vi "Video Detection.vi"() -> ()   [LabVIEW 2020]
doc: "Filtr detected objects and return only cars. Returns also the coordiantes of the nearest one."
uses:
  <vilib>/vision/Deep Learning.llb/IMAQ DL Model Type.ctl
  <vilib>/userDefined/High Color/IMAQdx.ctl
  <vilib>/vision/Avi.llb/IMAQ AVI2 Refnum.ctl
  <vilib>/vision/Avi.llb/IMAQ AVI2 Codec Path.ctl
  <vilib>/vision/Deep Learning.llb/IMAQ DL Model Detect Objects Node Names.ctl
  <vilib>/vision/Deep Learning.llb/IMAQ DL Model Label.ctl
  <vilib>/vision/NI_Vision_Development_Module.lvlib
  <vilib>/vision/driver/NI_Vision_Acquisition_Software.lvlib
  <resource>/objmgr/imaqdx.rc
panel:
  out "fps detection":dbl
  out "Replay mode":bool
  in  "Turn on the replay mode":bool
  in  "?":T1(tab)
  in  "Camera Name":refnum<k21> caption="IMAQdx Session"
  out "fps cam":dbl
  out "height":u32
  out "width":u32
  in  "Start Frame Number":u32
  out "Frame Number":u32
  in  "Frame increment":i32=1
  in  "Video fps":u32=30
  in  "Video filename":string="test_moving2.avi"
  in  "Height":i32=1080
  in  "Width":i32=1920
  out "Distance":sgl(graph)
  out "Cars found":i32
  out "Car found":bool
  in  "Minimum Score Threshold":sgl=0.3 min=0 max=1 step=0.1 format="%.3g"
  out "Actual frame":T2(plugin-control)
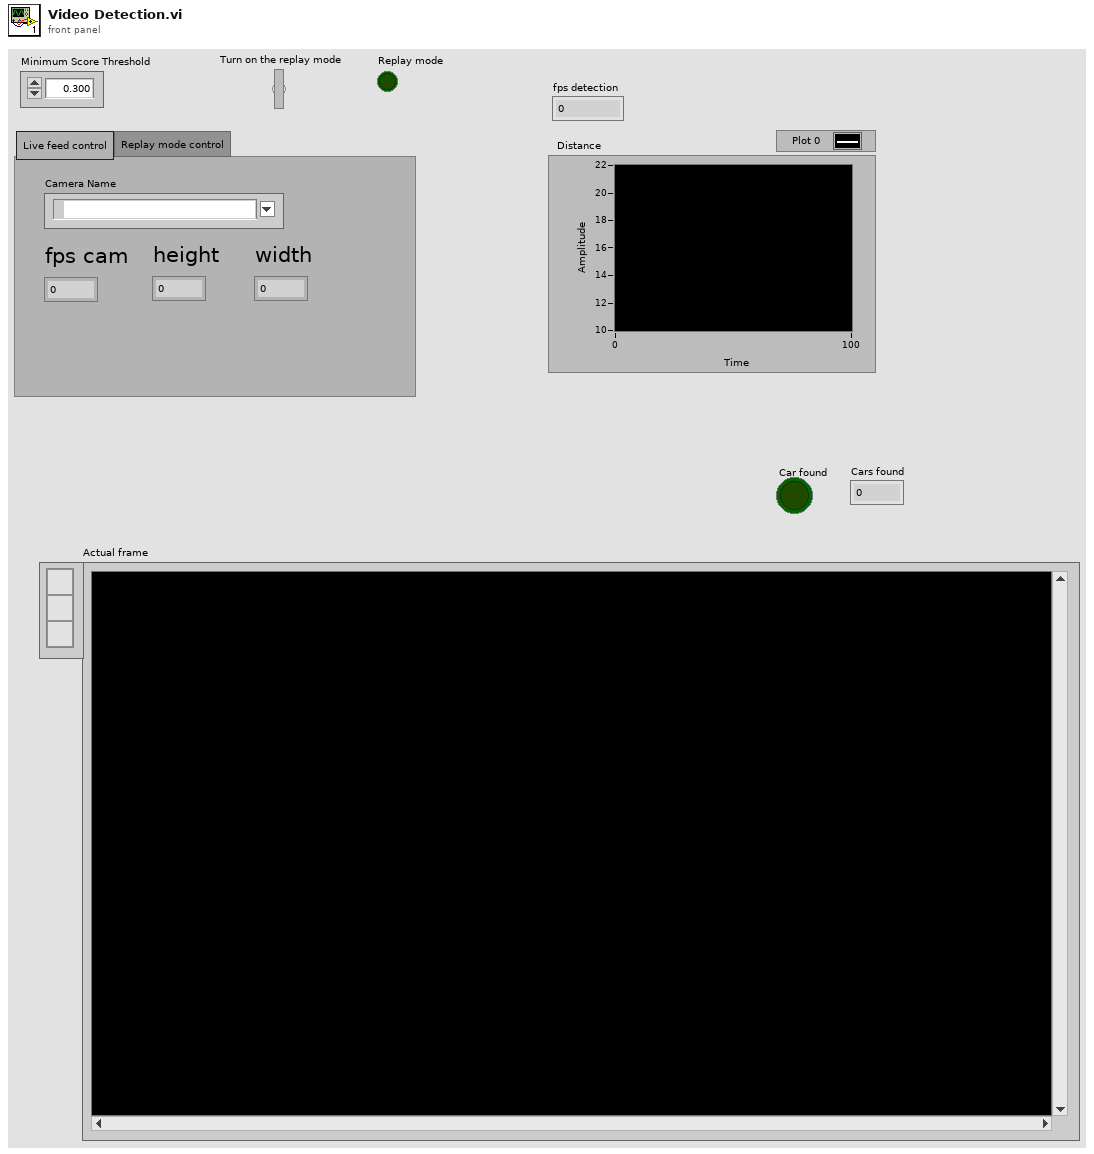
[diagram p1: front panel]
types:
  T1 = enum32{"Live feed control", "Replay mode control"}
  T2 = typedef "IMAQ Image.ctl" = refnum<image>
  T3 = typedef "IMAQdx.ctl" = refnum<k21>
  T4 = typedef "IMAQ AVI2 Refnum.ctl" = refnum<k20>
  T5 = typedef "IMAQ DL Model Type.ctl" = i32
  T6 = typedef "Image Type" = u32
  T7 = typedef "IMAQ AVI2 Codec Path.ctl" = u32
  T8 = typedef "IMAQ DL Model Refnum.ctl" = refnum<k20>
  T9 = typedef "IMAQ DL Model Label.ctl" = cluster{"ID":u32, "Label":string}
  T10 = typedef "IMAQ DL Model Detect Objects Node Names.ctl" = cluster{"Number of Objects":string, "Labels":string, "Scores":string, "Bounding Boxes":string}
  T11 = typedef "IMAQ DL Model Output Data.ctl" = cluster{"Node Name":string, "Data":sgl[], "Dimensions":u64[]}
  T12 = typedef "IMAQ DL Model Objects.ctl" = cluster{"Label":string, "Score":sgl, "Bounding Box":cluster{"x":sgl, "y":sgl}[]}
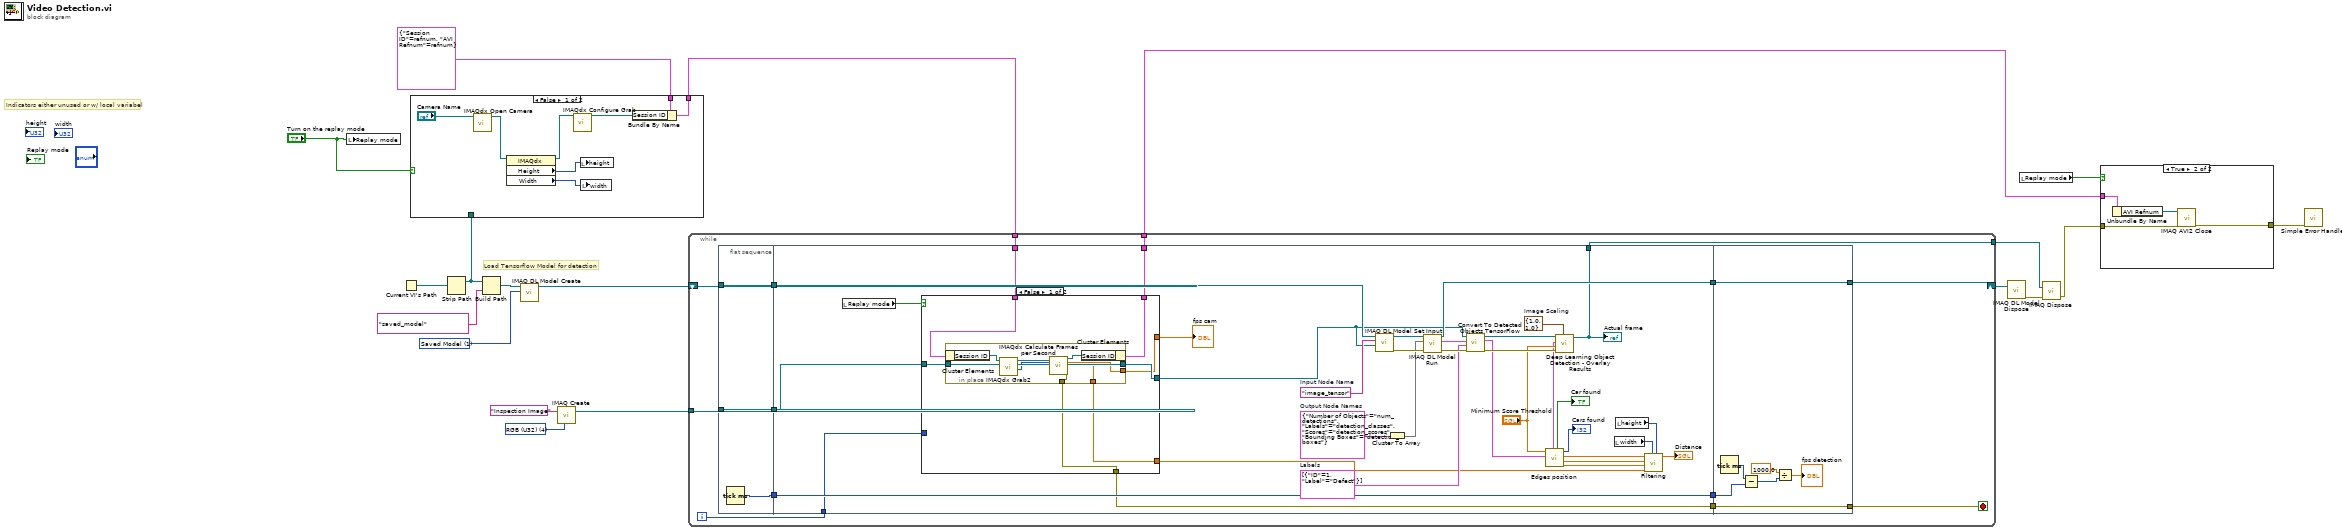
[diagram p0: block diagram]
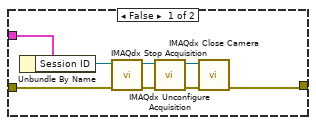
[diagram p2: hidden frame]
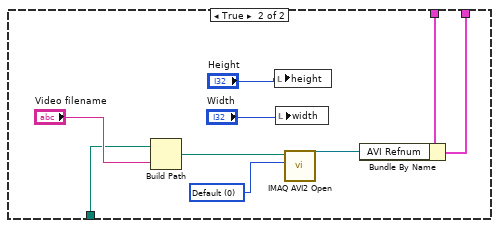
[diagram p3: hidden frame]
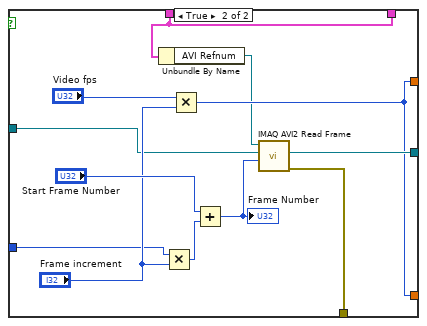
[diagram p4: hidden frame]
diagram:
  w12 = T5 1 items=["Frozen Graph", "Saved Model"] ("Model Type")
  w18 = T6 4 items=["Grayscale (U8)", "Grayscale (I16)", "Grayscale (SGL)", "Complex (CSG)", "RGB (U32)", "HSL (U32)", "RGB (U64)", "Grayscale (U16)"] ("Image Type")
  # "Indicators either unused or w/ local variabel"
  # "Load Tensorflow Model for detection"
  n1 = local write "Replay mode"("Turn on the replay mode") -> ()
  n2 = Current VI's Path() -> (path=w10:path)
  n3 = Strip Path(path=w10) -> (stripped path=w9:path)  [unwired: 1 out]
  n4 = case shown="False" "Turn on the replay mode" {
    tunnel: w9 -> [_ w33]
    tunnel: cluster{"Session ID":T3, "AVI Refnum":T4} {"Session ID"="", "AVI Refnum"=refnum} -> [w22 w30]
    tunnel: [w20 w28] -> w4
    frame False {
      n5 = call <vilib>:"IMAQdx Open Camera.vi"("Session In"="Camera Name") -> ("Session Out"=w26:T3)  [unwired: 2 in, 8 out]
      n6 = property class="IMAQdx"(reference=w26) -> (reference out=w27:T3, "Height"=w23:u32, "Width"=w24:u32)  [unwired: 1 in, 1 out]
      n7 = call <vilib>:"IMAQdx Configure Grab.vi"("Session In"=w27) -> ("Session Out"=w21:T3)  [unwired: 9 in, 1 out]
      n8 = local write "height"(w23) -> ()
      n9 = local write "width"(w24) -> ()
      n10 = Bundle By Name(cluster=w22, "Session ID"=w21) -> (w20:cluster{"Session ID":T3, "AVI Refnum":T4})
    }
    frame True {
      w36 = T7 0 items=["Default", "System", "Built in Vision"] ("Codec Source")
      n11 = Build Path(base path=w33, name or relative path="Video filename") -> (appended path=w35:path)
      n12 = local write "height"("Height") -> ()
      n13 = local write "width"("Width") -> ()
      n14 = call "IMAQ AVI2 Open"("Codec Source"=w36, "AVI File Path"=w35) -> ("AVI Refnum"=w29:T4)  [unwired: 8 in, 1 out]
      n15 = Bundle By Name(cluster=w30, "AVI Refnum"=w29) -> (w28:cluster{"Session ID":T3, "AVI Refnum":T4})
    }
  }
  n16 = Build Path(base path=w9, name or relative path="saved_model") -> (appended path=w14:path)
  n17 = call-poly "IMAQ DL Model Create"("Model Type"=w12, "File Path"=w14) -> ("Model Refnum"=w11:T8)  [unwired: 8 in, 1 out]
  n18 = call "IMAQ Create"("Image Name"="Inspection Image", "Image Type"=w18) -> ("New Image"=w16:T2)  [unwired: 3 in, 1 out]
  n19 = while {
    tunnel: w16 -> [w49]
    shift-right: [w48] -> w15
    shift-left: w11 -> [w50]
    tunnel: w4 -> [w39]
    tunnel: [w38] -> w3
    tunnel: [w37] -> w1
    i -> [w40]
    stop <- w47 stop-if-true
    n20 = flat-sequence {
      tunnel: w49 -> [w52]
      tunnel: w50 -> [w53]
      tunnel: [w53] -> w46
      tunnel: [w52] -> w45
      tunnel: [w51] -> w42
      tunnel: w46 -> [w77]
      tunnel: w45 -> [w68]
      tunnel: [w76] -> w44
      tunnel: [w67] -> w43
      tunnel: w42 -> [w70]
      tunnel: [w70] -> w41
      tunnel: w40 -> [w63]
      tunnel: w39 -> [w56]
      tunnel: [w55] -> w38
      tunnel: [w54] -> w37
      tunnel: [w122] -> w47
      tunnel: [w123] -> w48
      tunnel: w44 -> [w123]
      tunnel: w43 -> [w122]
      tunnel: w41 -> [w120]
      frame #0 {
        n21 = Tick Count (ms)() -> (millisecond timer value=w51:u32)
      }
      frame #1 {
        w79 = T9[] [{"ID"=1, "Label"="Defect"}]  # Labels
        w81 = T10 {"Number of Objects"="num_detections", "Labels"="detection_classes", "Scores"="detection_scores", "Bounding Boxes"="detection_boxes"}  # Output Node Names
        w87 = "image_tensor"  # Input Node Name
        w88 = cluster{"X":dbl, "Y":dbl} {"X"=1.0, "Y"=1.0}  # Image Scaling
        n22 = local read "Replay mode"() -> (w64:bool)
        n23 = case shown="False" w64 {
          tunnel: [w93 w111] -> w65
          tunnel: w68 -> [w94 w110]
          tunnel: [w91 w108] -> w62
          tunnel: [w90 w107] -> w67
          tunnel: [w92 w108] -> w66
          tunnel: w63 -> [_ w109]
          tunnel: w56 -> [w95 w105]
          tunnel: [w89 w105] -> w55
          frame False {
            n24 = in-place {
              in-place-border: w94 -> [w104]
              in-place-border: [w103] -> w93
              in-place-border: [w100] -> w92
              in-place-border: [w99] -> w91
              in-place-border: [w98] -> w90
              n25 = in-place-cluster #1(w95) -> ("Session ID"=w96:T3)
              n26 = call <vilib>:"IMAQdx Grab2.vi"("Image In"=w104, "Session In"=w96) -> ("Buffer Number Out"=w101:u32, "Image Out"=w103:T2, "Session Out"=w102:T3)  [unwired: 6 in, 1 out]
              n27 = call <vilib>:"IMAQdx Calculate Frames per Second.vi"("Session In"=w102, "Buffer Number"=w101) -> ("Session Out"=w97:T3, "Acquired Frames per Second"=w100:dbl, "Processed Frames per Second"=w99:dbl, "error out"=w98:errorcluster)  [unwired: 7 in, 3 out]
              n28 = in-place-cluster #1("Session ID"=w97) -> (w89:cluster{"Session ID":T3, "AVI Refnum":T4})
            }
          }
          frame True {
            n29 = Unbundle By Name(w105) -> ("AVI Refnum"=w106:T4)
            n30 = Multiply(x=w109, y="Frame increment") -> (x*y=w116:i32)
            n31 = Multiply(x="Video fps", y="Frame increment") -> (x*y=w108:u32)
            n32 = Add(x="Start Frame Number", y=w116) -> (x+y=w112:u32)
            "Frame Number" <- w112
            n33 = call "IMAQ AVI2 Read Frame"("Frame Number"=w112, "Image"=w110, "AVI Refnum"=w106) -> ("error out"=w107:errorcluster, "Image Out"=w111:T2)  [unwired: 6 in, 1 out]
          }
        }
        "fps cam" <- w66
        n34 = call-poly "IMAQ DL Model Set Input"("Image"=w65, "Input Node Name"=w87, "Model Refnum In"=w77) -> ("error out"=w85:errorcluster, "Model Refnum Out"=w86:T8)  [unwired: 6 in, 1 out]
        n35 = Cluster To Array(cluster=w81) -> (array=w80:string[])
        n36 = call "IMAQ DL Model Run"("error in (no error)"=w85, "Output Node Names"=w80, "Model Refnum In"=w86) -> ("error out"=w84:errorcluster, "Output Data Array"=w82:T11[], "Model Refnum Out"=w76:T8)  [unwired: 6 in]
        n37 = call "Convert To Detected Objects TensorFlow.vi"("error in (no error)"=w84, "Labels"=w79, "Output Data Array"=w82, "Image"=w65) -> ("error out"=w83:errorcluster, "Detected Objects"=w72:T12[], "Image (duplicate)"=w78:T2)  [unwired: 4 in, 1 out]
        n38 = call "Edges position.vi"("Detected Objects"=w72, "Minimum Score Threshold"="Minimum Score Threshold") -> ("bottom border"=w59:sgl, "left border"=w60:sgl, "right border"=w61:sgl, "Cars found"=→"Cars found":i32, "Car found"=→"Car found":bool, "nearest car object"=w71:T12[])  [unwired: 4 in]
        n39 = call "Deep Learning Object Detection - Overlay Results.vi"("Image Scaling"=w88, "error in (no error)"=w83, "Minimum Score Threshold"="Minimum Score Threshold", "Detected Objects"=w71, "Image In"=w78) -> ("Image Out"=w54:T2)  [unwired: 5 in, 1 out]
        "Actual frame" <- w54
        n40 = local read "width"() -> (w57:u32)
        n41 = local read "height"() -> (w58:u32)
        n42 = call "Filtering.vi"("Right border"=w61, "Left border"=w60, "Bottom border"=w59, "fps"=w62, "width"=w57, "height"=w58) -> ("distance"=→"Distance":sgl)  [unwired: 4 in]
      }
      frame #2 {
        n43 = Tick Count (ms)() -> (millisecond timer value=w121:u32)
        n44 = Subtract(x=w121, y=w120) -> (x-y=w118:u32)
        n45 = Divide(x=1000.0, y=w118) -> (x/y=→"fps detection":dbl)
      }
    }
  }
  n46 = call "IMAQ DL Model Dispose"("Model Refnum"=w15) -> ("error out"=w17:errorcluster)  [unwired: 10 in]
  n47 = local read "Replay mode"() -> (w6:bool)
  n48 = call "IMAQ Dispose"("Image"=w1, "error in (no error)"=w17) -> ("error out"=w8:errorcluster)  [unwired: 4 in]
  n49 = case shown="True" w6 {
    tunnel: w8 -> [w127 w135]
    tunnel: [w126 w134] -> w7
    tunnel: w3 -> [w125 w133]
    frame False {
      n50 = Unbundle By Name(w125) -> ("Session ID"=w124:T3)
      n51 = call <vilib>:"IMAQdx Stop Acquisition.vi"("error in"=w127, "Session In"=w124) -> ("error out"=w130:errorcluster, "Session Out"=w128:T3)  [unwired: 8 out]
      n52 = call <vilib>:"IMAQdx Unconfigure Acquisition.vi"("error in"=w130, "Session In"=w128) -> ("error out"=w131:errorcluster, "Session Out"=w129:T3)  [unwired: 8 out]
      n53 = call <vilib>:"IMAQdx Close Camera.vi"("error in"=w131, "Session In"=w129) -> ("error out"=w126:errorcluster)  [unwired: 9 out]
    }
    frame True {
      n54 = Unbundle By Name(w133) -> ("AVI Refnum"=w132:T4)
      n55 = call "IMAQ AVI2 Close"("error in (no error)"=w135, "AVI Refnum"=w132) -> ("error out"=w134:errorcluster)  [unwired: 9 in]
    }
  }
  n56 = call <vilib>:"Simple Error Handler.vi"("error in (no error)"=w7) -> ()  [unwired: 4 in, 5 out]
